vi "ContourPlot v4.5 IV.vi"() -> ()   [LabVIEW 2020]
uses:
  diff para.ctl
  graph para.ctl
  <vilib>/Analysis/NI_AALPro.lvlib
  <vilib>/gmath/NI_Gmath.lvlib
panel:
  out "Field data":dbl[](array[numeric])
  in  "Help":bool caption="load data"
  out "smoothed dIV buffer":dbl[][](array[numeric])
  in  "diff para":T1={"x0"=-1.0, "Ic0"=2.0, "h0"=1.0, "y0"=0.0}
  in  "Plot reference":bool caption="load data"
  out "smoothed dIV":dbl[][](array[numeric])
  out "smoothed data":dbl[][](array[numeric])
  in  "smooth n":i32=10
  out "IVdata":dbl[][](array[numeric])
  in  "load data":bool
  out "Status":string="Stopped"
  in  "stop":bool
  in  "Begin":i32=2000
  in  "length":i32=2000
  in  "Contact Resistance":dbl
  in  "Tab Control 2":enum32{"IV plots", "IV smoothed", "dV/dI"}(tab)=enum."dV/dI"
  in  "extract contour":bool caption="load data"
  out "IV Intensity":dbl[][](graph)
  out "IV":T2(graph)
  in  "polynomial order":i32=22
  out "Contour":cluster{"Field data":dbl[], dbl[]}(graph)
  in  "Threshold":dbl
  in  "Plot contour line":bool
  out "IV smoothed intensity":dbl[][](graph)
  out "Smooth IV":cluster{dbl[], "Intensity Graph":dbl[]}(graph)
  in  "Set diff parameter":bool caption="load data"
  out "dVdI Intensity":dbl[][](graph)
  out "dV/dI":cluster{dbl[], "Intensity Graph":dbl[]}(graph)
  in  "book number":i32=703
  in  "file path":path
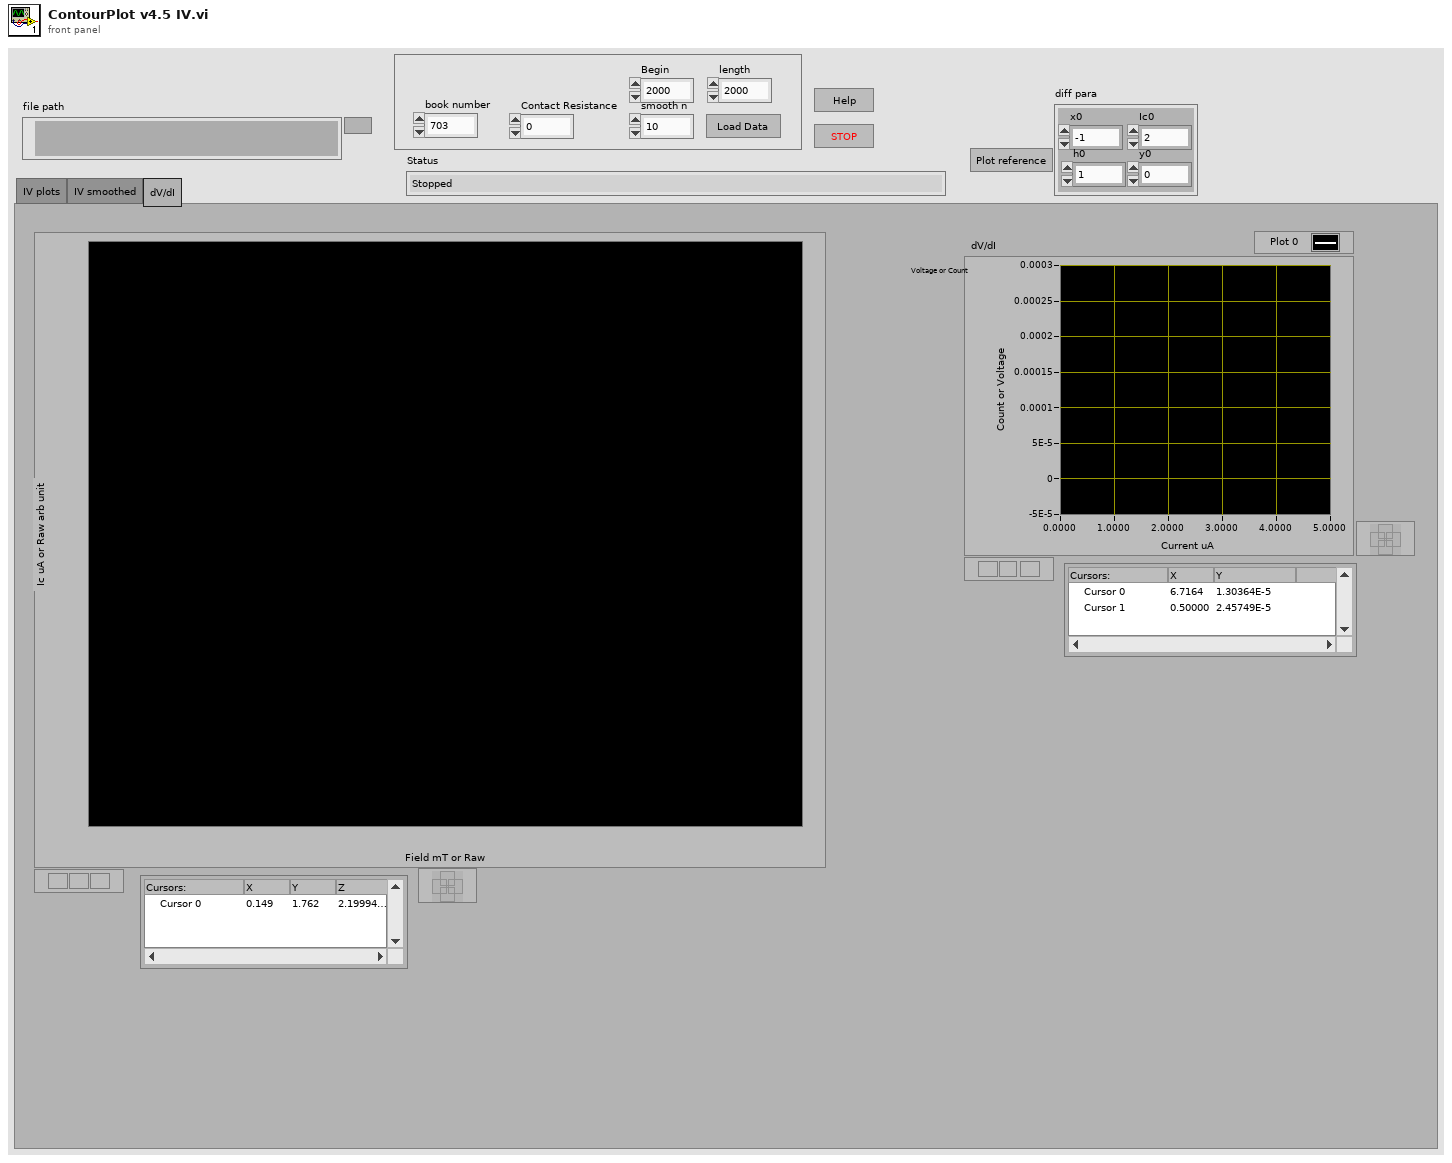
[diagram p1: front panel]
types:
  T1 = typedef "diff para.ctl" = cluster{"x0":dbl, "Ic0":dbl, "h0":dbl, "y0":dbl}
  T2 = cluster{"X":dbl[], "Best Polynomial Fit":dbl[]}[]
  T3 = typedef "graph para.ctl" = cluster{"x offset":dbl, "y offset":dbl, "x scale":dbl, "y scale":dbl}
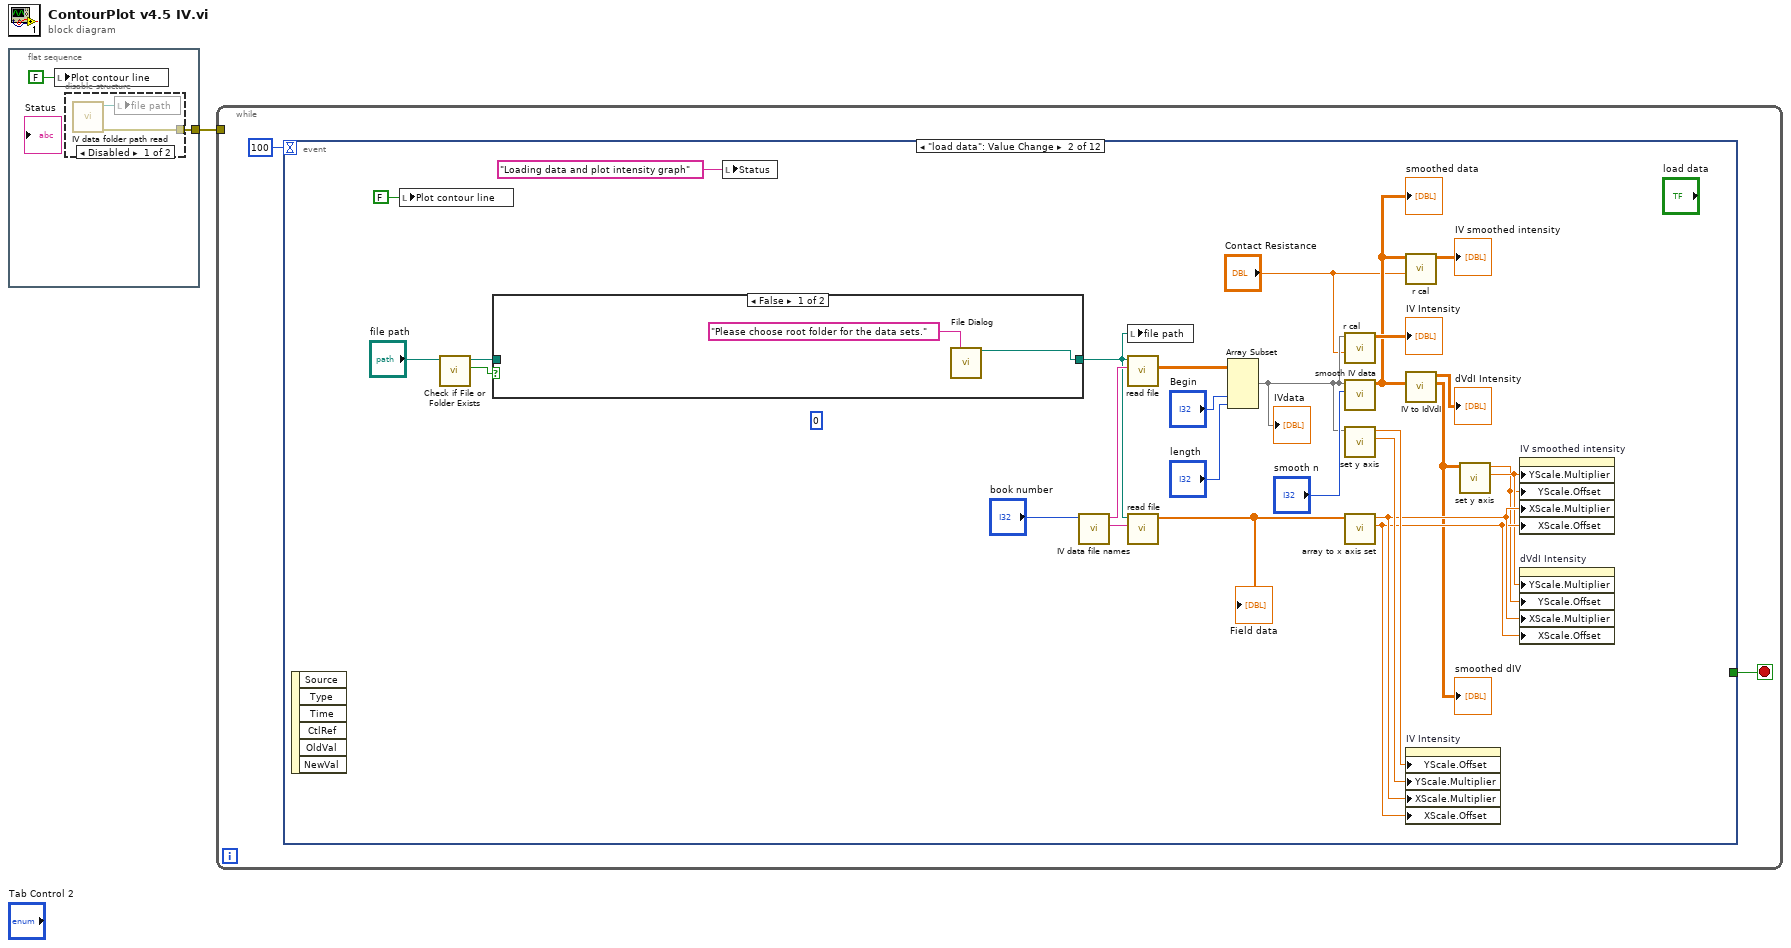
[diagram p0: block diagram]
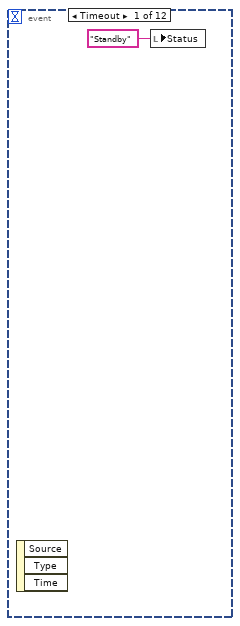
[diagram p3: hidden frame]
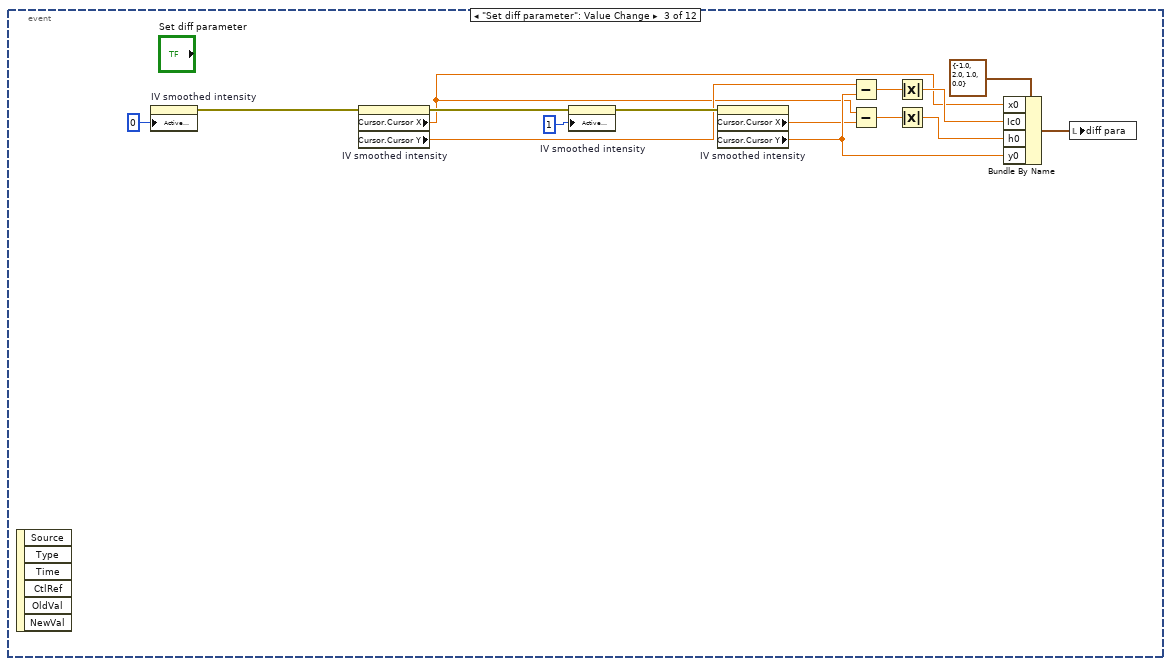
[diagram p5: hidden frame]
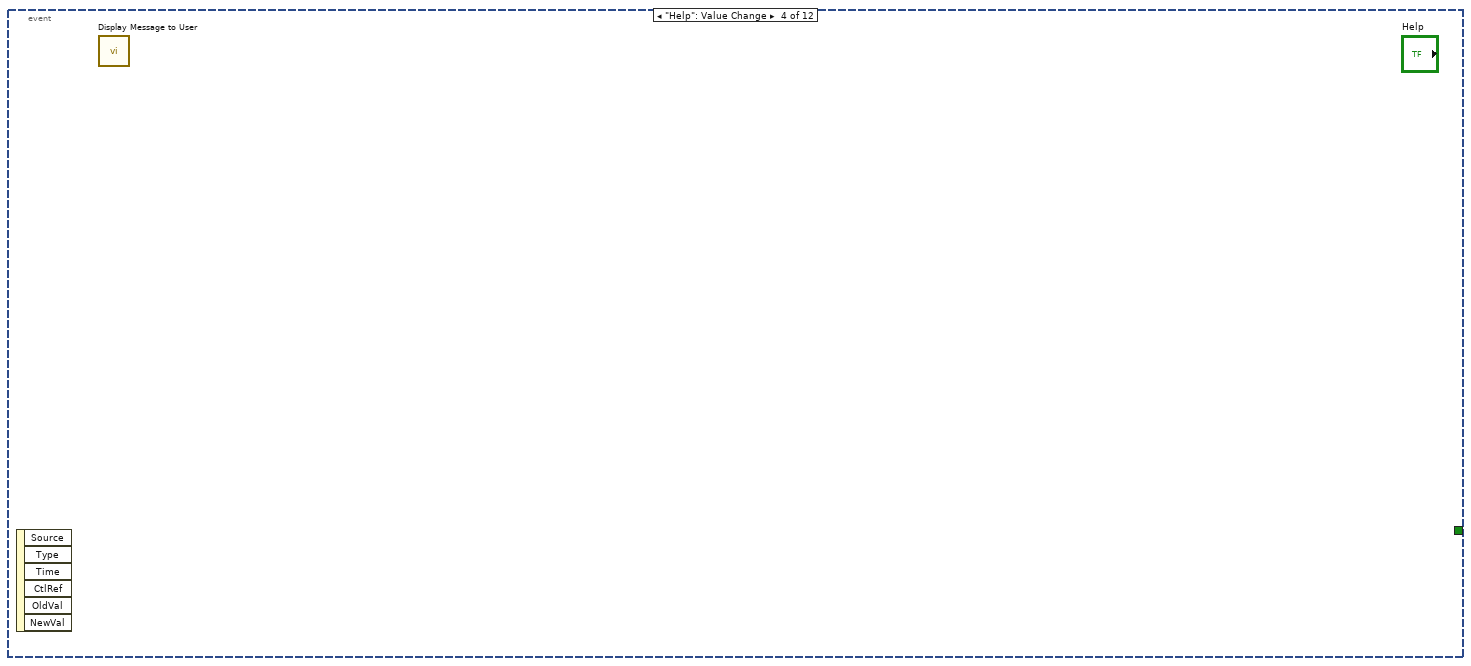
[diagram p6: hidden frame]
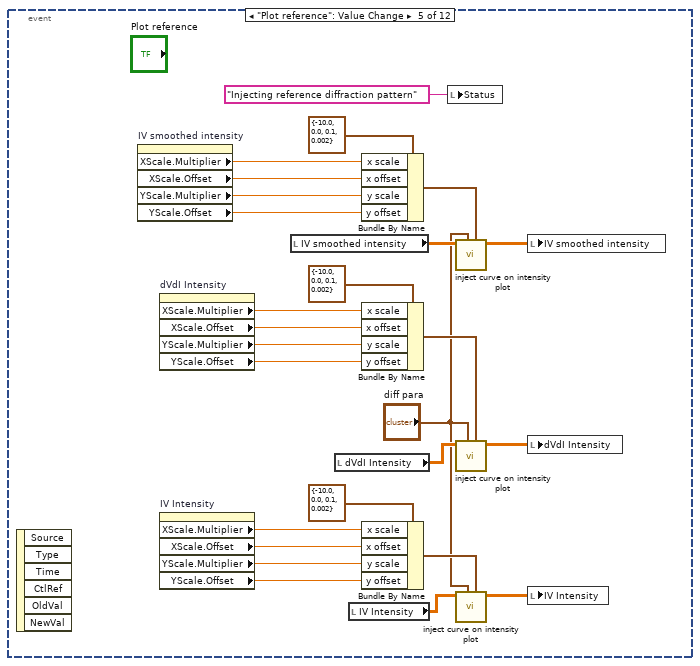
[diagram p7: hidden frame]
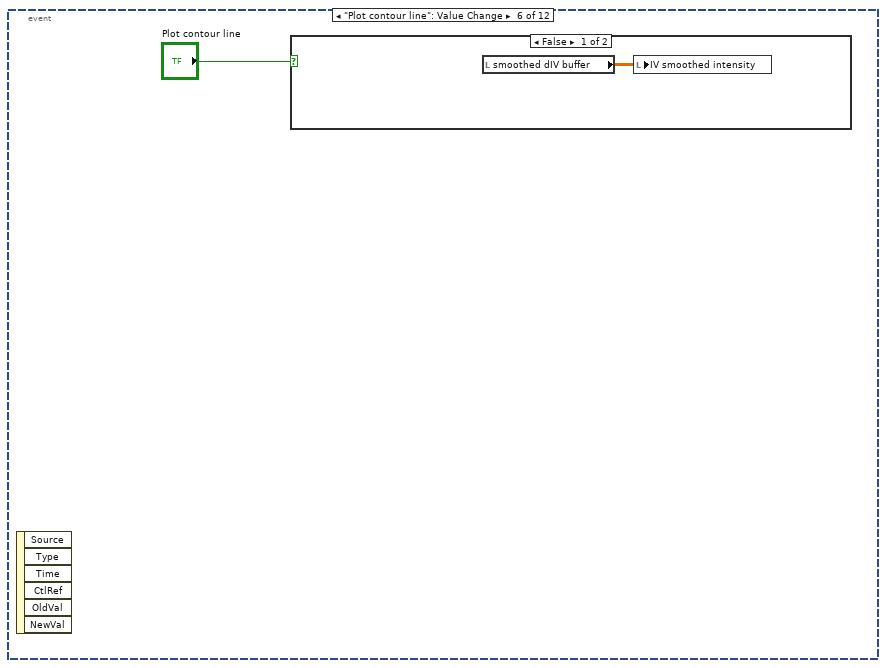
[diagram p8: hidden frame]
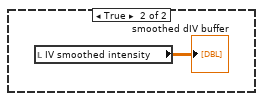
[diagram p9: hidden frame]
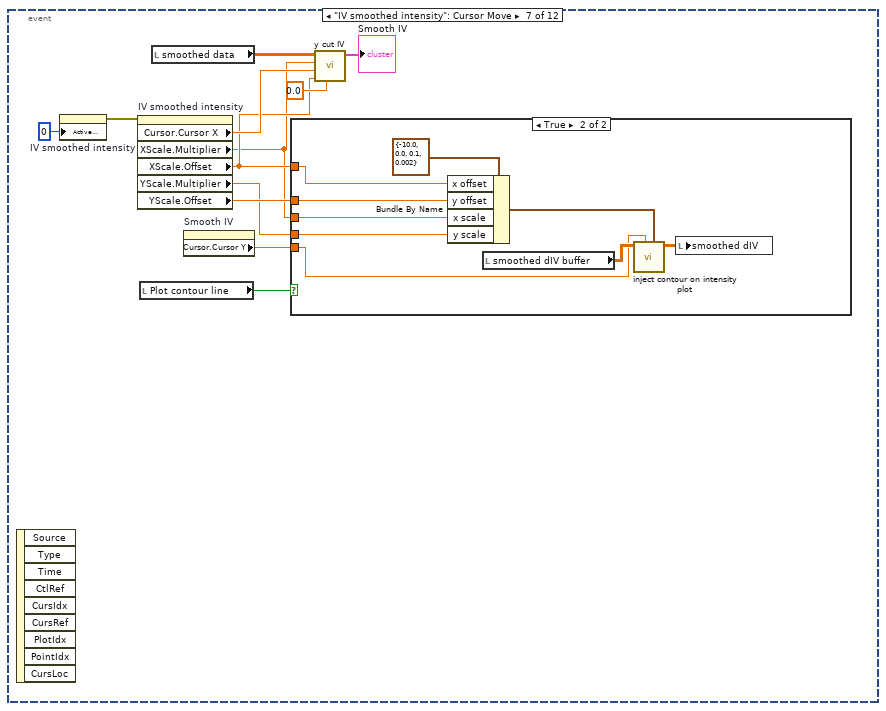
[diagram p10: hidden frame]
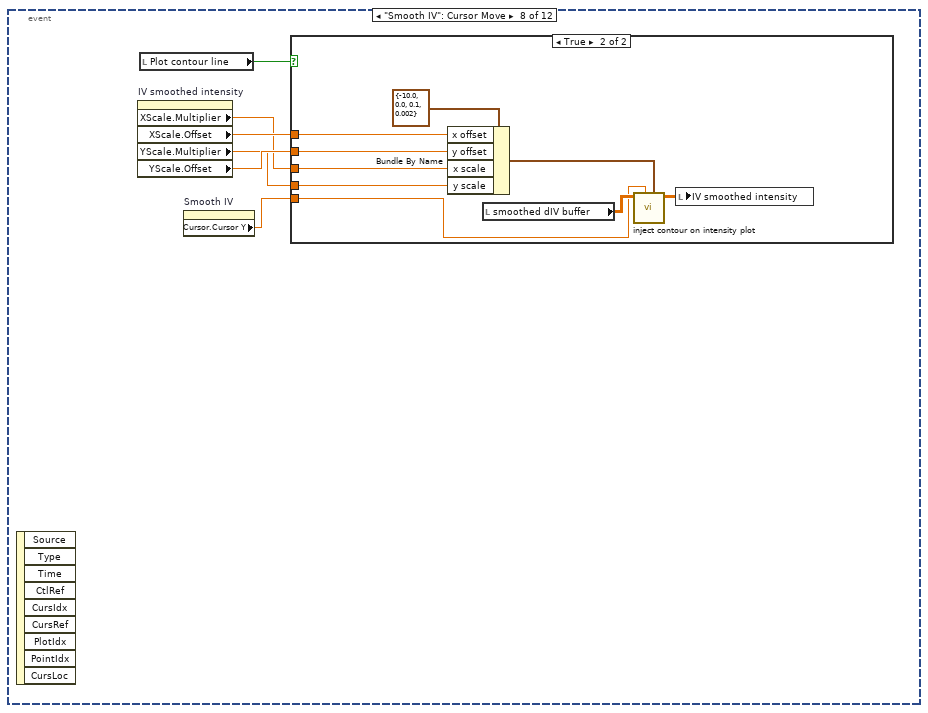
[diagram p12: hidden frame]
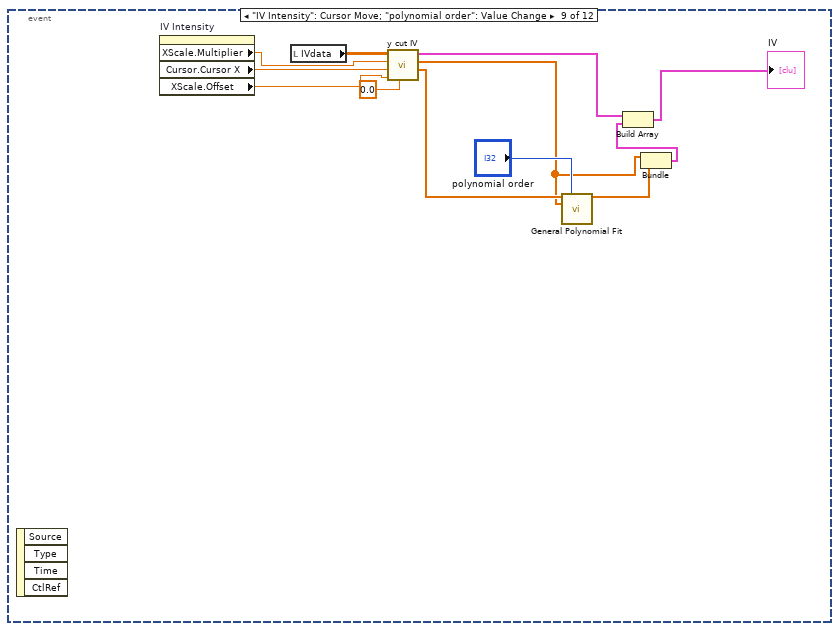
[diagram p14: hidden frame]
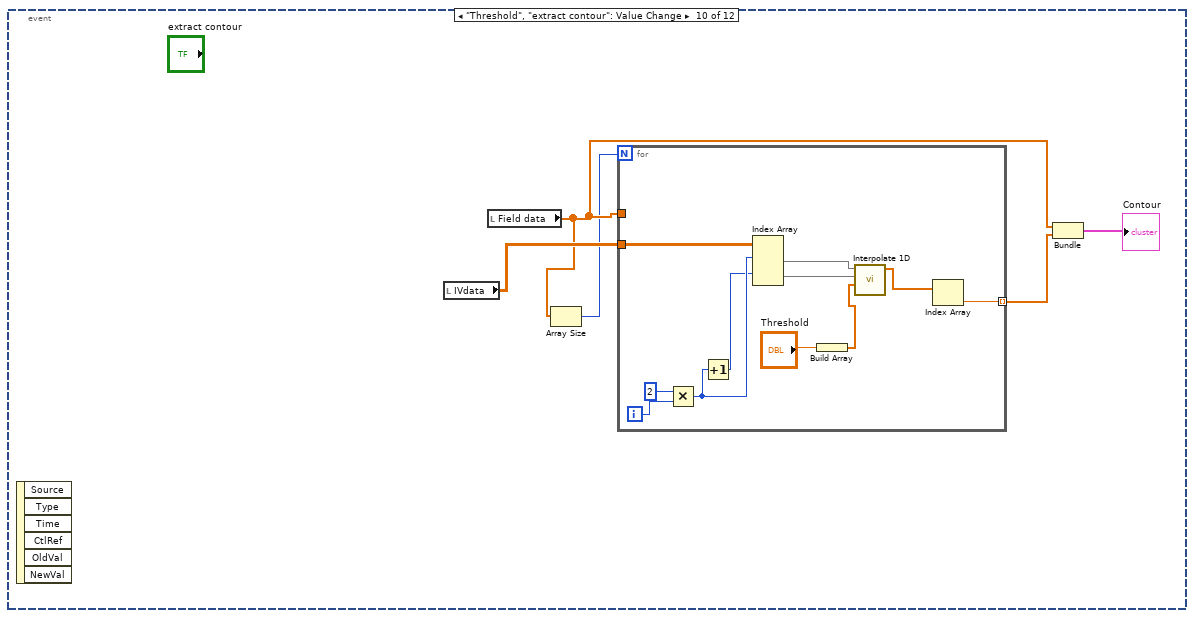
[diagram p15: hidden frame]
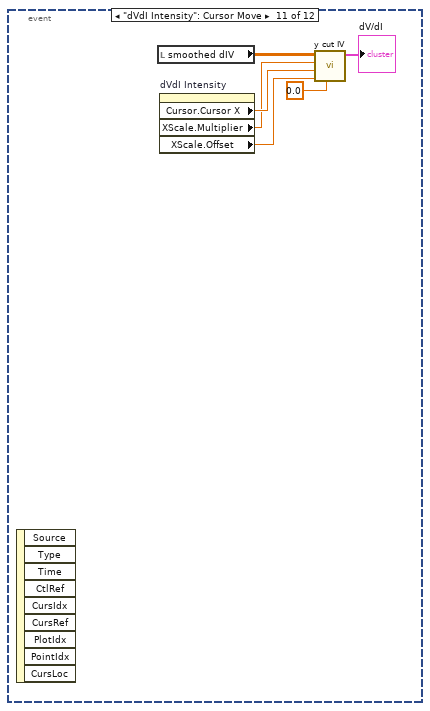
[diagram p16: hidden frame]
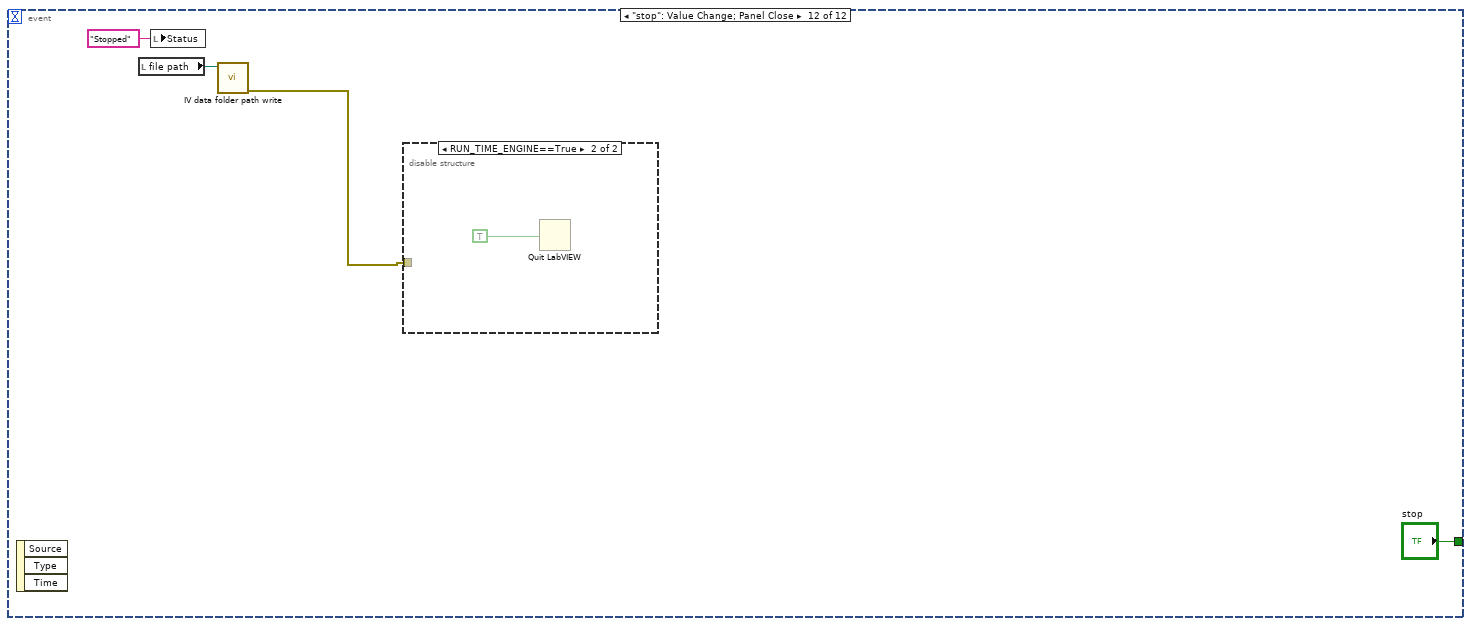
[diagram p17: hidden frame]
diagram:
  n1 = flat-sequence {
    tunnel: [w2] -> w1
    frame #0 {
      n2 = local write "Plot contour line"(FALSE ("Plot contour line")) -> ()
      n3 = disable-structure shown="Disabled" {
        disable-tunnel: [w4 _] -> w2
        frame Disabled {
          n4 = call "IV data folder path read.vi"() -> ("error out"=w4:errorcluster, "path"=w5:path)  [unwired: 10 in]
          n5 = local write "file path"(w5) -> ()
        }
        frame Enabled {
        }
      }
    }
  }
  n6 = while {
    tunnel: w1 -> [_]
    stop <- w6 stop-if-true
    n7 = event shown="[1] \"load data\": Value Change" {
      selector: _ -> [_ _ _ _ _ _ _ _ _ _ _ _]
      dyn-events: _ -> [_ _ _ _ _ _ _ _ _ _ _ _]
      timeout: 100 -> [_ _ _ _ _ _ _ _ _ _ _ _]
      tunnel: [_ _ _ _ _ _ _ _ _ _ _ "stop"] -> w6
      event Timeout {
        n8 = event-data() -> ()  [unwired: 1 in, 3 out]
        n9 = local write "Status"("Standby" ("Status")) -> ()
      }
      event "load data": Value Change {
        (unwired) 0 ("index (row)")
        n10 = event-data() -> ()  [unwired: 1 in, 6 out]
        n11 = local write "Plot contour line"(FALSE ("Plot contour line")) -> ()
        n12 = call <vilib>:"Check if File or Folder Exists.vi"("path"="file path") -> ("file or folder exists?"=w11:bool, "dup path"=w10:path)  [unwired: 8 in, 1 out]
        n13 = case shown="False" w11 {
          tunnel: [w36 w38] -> w9
          tunnel: w10 -> [_ w38]
          frame False {
            n14 = call "File Dialog"("prompt"="Please choose root folder for the data sets.") -> ("selected path"=w36:path)  [unwired: 11 in, 3 out]
          }
          frame True {
          }
        }
        n15 = local write "Status"("Loading data and plot intensity graph" ("Status")) -> ()
        n16 = call "IV data file names.vi"("book number"="book number") -> ("Field"=w34:string, "IV"=w33:string)  [unwired: 8 in, 1 out]
        n17 = local write "file path"(w9) -> ()
        n18 = call "read file.vi"("file name"=w33, "file path (dialog if empty)"=w9) -> ("2d data"=w26:dbl[][])  [unwired: 8 in, 1 out]
        n19 = call "read file.vi"("file name"=w34, "file path (dialog if empty)"=w9) -> ("1d Data"=w25:dbl[])  [unwired: 8 in, 1 out]
        "Field data" <- w25
        n20 = Array Subset(array=w26, index (col)="Begin", length (col)="length") -> (w22:dbl[][])  [unwired: 2 in]
        "IVdata" <- w22
        n21 = call "r cal.vi"("Contact Resistance"="Contact Resistance", "Array in"=w22) -> ("Array out"=→"IV Intensity":dbl[][])  [unwired: 9 in]
        n22 = call "smooth IV data.vi"("smooth n"="smooth n", "Array in"=w22) -> ("Array out"=w21:dbl[][])  [unwired: 9 in]
        "smoothed data" <- w21
        n23 = call "set y axis.vi"("Array"=w22) -> ("y multi"=w32:dbl, "y offset"=w31:dbl)  [unwired: 9 in]
        n24 = call "array to x axis set.vi"("1d Data"=w25) -> ("offset"=w17:dbl, "multiplier"=w18:dbl)  [unwired: 9 in]
        n25 = call "r cal.vi"("Contact Resistance"="Contact Resistance", "Array in"=w21) -> ("Array out"=→"IV smoothed intensity":dbl[][])  [unwired: 9 in]
        n26 = call "IV to IdVdI.vi"("Array in"=w21) -> ("Array"=w16:dbl[][], "Array 2"=→"dVdI Intensity":dbl[][])  [unwired: 9 in]
        "smoothed dIV" <- w16
        n27 = property on="IV Intensity" class="IntGraph (strict)"("YScale.Offset"=w31, "YScale.Multiplier"=w32, "XScale.Multiplier"=w18, "XScale.Offset"=w17) -> ()  [unwired: 2 in, 2 out]
        n28 = call "set y axis.vi"("Array"=w16) -> ("y multi"=w15:dbl, "y offset"=w14:dbl)  [unwired: 9 in]
        n29 = property on="IV smoothed intensity" class="IntGraph (strict)"("YScale.Multiplier"=w15, "YScale.Offset"=w14, "XScale.Multiplier"=w18, "XScale.Offset"=w17) -> ()  [unwired: 2 in, 2 out]
        n30 = property on="dVdI Intensity" class="IntGraph (strict)"("YScale.Multiplier"=w15, "YScale.Offset"=w14, "XScale.Multiplier"=w18, "XScale.Offset"=w17) -> ()  [unwired: 2 in, 2 out]
      }
      event "Set diff parameter": Value Change {
        n31 = event-data() -> ()  [unwired: 1 in, 6 out]
        n32 = property on="IV smoothed intensity" class="IntGraph (strict)"("Active Cursor"=u32 0) -> (error out=w53:errorcluster)  [unwired: 2 in, 1 out]
        n33 = property on="IV smoothed intensity" class="IntGraph (strict)"(error in=w53) -> (error out=w50:errorcluster, "Cursor.Cursor X"=w42:dbl, "Cursor.Cursor Y"=w46:dbl)  [unwired: 1 in, 1 out]
        n34 = property on="IV smoothed intensity" class="IntGraph (strict)"(error in=w50, "Active Cursor"=u32 1) -> (error out=w49:errorcluster)  [unwired: 1 in, 1 out]
        n35 = property on="IV smoothed intensity" class="IntGraph (strict)"(error in=w49) -> ("Cursor.Cursor X"=w41:dbl, "Cursor.Cursor Y"=w45:dbl)  [unwired: 1 in, 2 out]
        n36 = Subtract(x=w46, y=w45) -> (x-y=w44:dbl)
        n37 = Subtract(x=w42, y=w41) -> (x-y=w40:dbl)
        n38 = Absolute Value(x=w44) -> (abs(x)=w43:dbl)
        n39 = Absolute Value(x=w40) -> (abs(x)=w39:dbl)
        n40 = Bundle By Name(cluster=T1 {"x0"=-1.0, "Ic0"=2.0, "h0"=1.0, "y0"=0.0} ("diff para"), "x0"=w42, "Ic0"=w43, "h0"=w39, "y0"=w45) -> (w48:T1)
        n41 = local write "diff para"(w48) -> ()
      }
      event "Help": Value Change {
        n42 = event-data() -> ()  [unwired: 1 in, 6 out]
        n43 = call "Display Message to User"() -> ()  [unwired: 10 in, 2 out]
      }
      event "Plot reference": Value Change {
        n44 = event-data() -> ()  [unwired: 1 in, 6 out]
        n45 = property on="IV smoothed intensity" class="IntGraph (strict)"() -> ("XScale.Multiplier"=w65:dbl, "XScale.Offset"=w64:dbl, "YScale.Multiplier"=w63:dbl, "YScale.Offset"=w62:dbl)  [unwired: 2 in, 2 out]
        n46 = property on="dVdI Intensity" class="IntGraph (strict)"() -> ("XScale.Multiplier"=w59:dbl, "XScale.Offset"=w58:dbl, "YScale.Multiplier"=w57:dbl, "YScale.Offset"=w56:dbl)  [unwired: 2 in, 2 out]
        n47 = property on="IV Intensity" class="IntGraph (strict)"() -> ("XScale.Multiplier"=w77:dbl, "XScale.Offset"=w76:dbl, "YScale.Multiplier"=w75:dbl, "YScale.Offset"=w74:dbl)  [unwired: 2 in, 2 out]
        n48 = local read "IV smoothed intensity"() -> (w66:dbl[][])
        n49 = local read "dVdI Intensity"() -> (w60:dbl[][])
        n50 = local read "IV Intensity"() -> (w79:dbl[][])
        n51 = Bundle By Name(cluster=T3 {"x offset"=-10.0, "y offset"=0.0, "x scale"=0.1, "y scale"=0.002} ("graph para"), "x scale"=w65, "x offset"=w64, "y scale"=w63, "y offset"=w62) -> (w69:T3)
        n52 = Bundle By Name(cluster=T3 {"x offset"=-10.0, "y offset"=0.0, "x scale"=0.1, "y scale"=0.002} ("graph para"), "x scale"=w59, "x offset"=w58, "y scale"=w57, "y offset"=w56) -> (w67:T3)
        n53 = Bundle By Name(cluster=T3 {"x offset"=-10.0, "y offset"=0.0, "x scale"=0.1, "y scale"=0.002} ("graph para"), "x scale"=w77, "x offset"=w76, "y scale"=w75, "y offset"=w74) -> (w73:T3)
        n54 = local write "Status"("Injecting reference diffraction pattern" ("Status")) -> ()
        n55 = call "inject curve on intensity plot.vi"("graph para"=w69, "diff para"="diff para", "IV Intensity"=w66) -> ("IV Intensity 2"=w61:dbl[][])  [unwired: 8 in]
        n56 = call "inject curve on intensity plot.vi"("graph para"=w67, "diff para"="diff para", "IV Intensity"=w60) -> ("IV Intensity 2"=w54:dbl[][])  [unwired: 8 in]
        n57 = call "inject curve on intensity plot.vi"("graph para"=w73, "diff para"="diff para", "IV Intensity"=w79) -> ("IV Intensity 2"=w72:dbl[][])  [unwired: 8 in]
        n58 = local write "IV smoothed intensity"(w61) -> ()
        n59 = local write "dVdI Intensity"(w54) -> ()
        n60 = local write "IV Intensity"(w72) -> ()
      }
      event "Plot contour line": Value Change {
        n61 = event-data() -> ()  [unwired: 1 in, 6 out]
        n62 = case shown="False" "Plot contour line" {
          frame False {
            n63 = local read "smoothed dIV buffer"() -> (w81:dbl[][])
            n64 = local write "IV smoothed intensity"(w81) -> ()
          }
          frame True {
            n65 = local read "IV smoothed intensity"() -> (→"smoothed dIV buffer":dbl[][])
          }
        }
      }
      event "IV smoothed intensity": Cursor Move {
        n66 = event-data() -> ()  [unwired: 1 in, 9 out]
        n67 = property on="IV smoothed intensity" class="IntGraph (strict)"("Active Cursor"=u32 0) -> (error out=w83:errorcluster)  [unwired: 2 in, 1 out]
        n68 = property on="IV smoothed intensity" class="IntGraph (strict)"(error in=w83) -> ("Cursor.Cursor X"=w91:dbl, "XScale.Multiplier"=w87:dbl, "XScale.Offset"=w89:dbl, "YScale.Multiplier"=w86:dbl, "YScale.Offset"=w88:dbl)  [unwired: 1 in, 2 out]
        n69 = local read "Plot contour line"() -> (w90:bool)
        n70 = local read "smoothed data"() -> (w94:dbl[][])
        n71 = property on="Smooth IV" class="XYGraph (strict)"() -> ("Cursor.Cursor Y"=w85:dbl)  [unwired: 2 in, 2 out]
        n72 = case shown="True" w90 {
          tunnel: w85 -> [_ w101]
          tunnel: w89 -> [_ w99]
          tunnel: w88 -> [_ w98]
          tunnel: w87 -> [_ w97]
          tunnel: w86 -> [_ w96]
          frame False {
          }
          frame True {
            n73 = Bundle By Name(cluster=T3 {"x offset"=-10.0, "y offset"=0.0, "x scale"=0.1, "y scale"=0.002} ("graph para"), "x offset"=w99, "y offset"=w98, "x scale"=w97, "y scale"=w96) -> (w95:T3)
            n74 = local read "smoothed dIV buffer"() -> (w103:dbl[][])
            n75 = call "inject contour on intensity plot.vi"("graph para"=w95, "Threshold"=w101, "IV Intensity"=w103) -> ("IV Intensity output"=w102:dbl[][])  [unwired: 6 in, 2 out]
            n76 = local write "smoothed dIV"(w102) -> ()
          }
        }
        n77 = call "y cut IV.vi"("Contact Resistance"=0.0, "x offset"=w89, "x pos"=w91, "scale"=w87, "Data"=w94) -> ("IV"=→"Smooth IV":cluster{"Data":dbl[], dbl[]})  [unwired: 4 in, 2 out]
      }
      event "Smooth IV": Cursor Move {
        n78 = event-data() -> ()  [unwired: 1 in, 9 out]
        n79 = property on="IV smoothed intensity" class="IntGraph (strict)"() -> ("XScale.Multiplier"=w106:dbl, "XScale.Offset"=w108:dbl, "YScale.Multiplier"=w105:dbl, "YScale.Offset"=w107:dbl)  [unwired: 2 in, 2 out]
        n80 = local read "Plot contour line"() -> (w109:bool)
        n81 = property on="Smooth IV" class="XYGraph (strict)"() -> ("Cursor.Cursor Y"=w104:dbl)  [unwired: 2 in, 2 out]
        n82 = case shown="True" w109 {
          tunnel: w104 -> [_ w116]
          tunnel: w108 -> [_ w114]
          tunnel: w107 -> [_ w113]
          tunnel: w106 -> [_ w112]
          tunnel: w105 -> [_ w111]
          frame False {
          }
          frame True {
            n83 = Bundle By Name(cluster=T3 {"x offset"=-10.0, "y offset"=0.0, "x scale"=0.1, "y scale"=0.002} ("graph para"), "x offset"=w114, "y offset"=w113, "x scale"=w112, "y scale"=w111) -> (w110:T3)
            n84 = local read "smoothed dIV buffer"() -> (w118:dbl[][])
            n85 = call "inject contour on intensity plot.vi"("graph para"=w110, "Threshold"=w116, "IV Intensity"=w118) -> ("IV Intensity output"=w117:dbl[][])  [unwired: 6 in, 2 out]
            n86 = local write "IV smoothed intensity"(w117) -> ()
          }
        }
      }
      event "IV Intensity": Cursor Move; "polynomial order": Value Change {
        n87 = event-data() -> ()  [unwired: 1 in, 4 out]
        n88 = property on="IV Intensity" class="IntGraph (strict)"() -> ("XScale.Multiplier"=w128:dbl, "Cursor.Cursor X"=w129:dbl, "XScale.Offset"=w130:dbl)  [unwired: 2 in, 2 out]
        n89 = local read "IVdata"() -> (w127:dbl[][])
        n90 = call "y cut IV.vi"("Contact Resistance"=0.0, "x offset"=w130, "x pos"=w129, "scale"=w128, "Data"=w127) -> ("Y"=w124:dbl[], "X"=w122:dbl[], "IV"=w123:cluster{"Data":dbl[], dbl[]})  [unwired: 4 in]
        n91 = call <vilib>:"General Polynomial Fit.vi"("Y"=w124, "polynomial order"="polynomial order", "X"=w122) -> ("Best Polynomial Fit"=w121:dbl[])  [unwired: 9 in, 3 out]
        n92 = Bundle("X"=w122, "Best Polynomial Fit"=w121) -> (w120:cluster{"X":dbl[], "Best Polynomial Fit":dbl[]})  [unwired: 1 in]
        n93 = Build Array(w123, w120) -> (→"IV":T2)
      }
      event "Threshold", "extract contour": Value Change {
        n94 = event-data() -> ()  [unwired: 1 in, 6 out]
        n95 = local read "IVdata"() -> (w134:dbl[][])
        n96 = local read "Field data"() -> (w132:dbl[])
        n97 = Array Size(array=w132) -> (size(s)=w131:i32)
        n98 = for {
          N: w131 -> [_]
          tunnel: w132 -> [_]
          tunnel: w134 -> [w144]
          tunnel: [w136] -> w133 mode=indexing
          i -> [w146]
          n99 = Multiply(x=2, y=w146) -> (x*y=w143:i32)
          n100 = Increment(x=w143) -> (x+1=w142:i32)
          n101 = Index Array(array=w144, index (row) #1=w143, index (row) #2=w142) -> (element #1=w141:dbl[], element #2=w140:dbl[])  [unwired: 2 in]
          n102 = Build Array("Threshold") -> (w138:dbl[])
          n103 = call <vilib>:"Interpolate 1D.vi"("xi"=w138, "X"=w140, "Y"=w141) -> ("yi"=w137:dbl[])  [unwired: 6 in, 2 out]
          n104 = Index Array(array=w137) -> (element=w136:dbl)  [unwired: 1 in]
        }
        n105 = Bundle("Field data"=w132, w133) -> (→"Contour":cluster{"Field data":dbl[], dbl[]})  [unwired: 1 in]
      }
      event "dVdI Intensity": Cursor Move {
        n106 = event-data() -> ()  [unwired: 1 in, 9 out]
        n107 = local read "smoothed dIV"() -> (w152:dbl[][])
        n108 = property on="dVdI Intensity" class="IntGraph (strict)"() -> ("Cursor.Cursor X"=w150:dbl, "XScale.Multiplier"=w149:dbl, "XScale.Offset"=w148:dbl)  [unwired: 2 in, 2 out]
        n109 = call "y cut IV.vi"("Contact Resistance"=0.0, "x offset"=w148, "x pos"=w150, "scale"=w149, "Data"=w152) -> ("IV"=→"dV/dI":cluster{"Data":dbl[], dbl[]})  [unwired: 4 in, 2 out]
      }
      event "stop": Value Change; Panel Close {
        n110 = event-data() -> ()  [unwired: 1 in, 3 out]
        n111 = local read "file path"() -> (w154:path)
        n112 = local write "Status"("Stopped" ("Status")) -> ()
        n113 = call "IV data folder path write.vi"("Path"=w154) -> ("error out"=w153:errorcluster)  [unwired: 10 in]
        n114 = disable-structure shown="RUN_TIME_ENGINE==True" {
          disable-tunnel: w153 -> [_ _]
          frame condition #0 (active) {
          }
          frame condition #1 {
            n115 = Quit LabVIEW(quit? (T)=TRUE) -> ()
          }
        }
      }
    }
  }
